vi "2D history.vi"   [LabVIEW 2021, in "Ring Buffer Strict Accessor Unit Tests.lvlib"]
uses:
  Ring Buffer Strict Accessor Unit Tests.lvlib
  Source/SubVIs/Endianess.ctl
  5a55b556-92d1-451c-b900-68450bc60f93.vi
  f229ef0f-1417-44bb-8496-cd9db5c3eb53.vi
  1447380f-0aa4-4579-b3fa-dda44ae90fdf.vi
  790f1047-96a1-4b40-bfa0-34b754fa4794.vi
  d13a2722-8c13-4299-92d3-41a30a9094d1.vi
  b8cc0c8d-ce30-4fd4-b064-991c88513f8d.vi
  ae355991-2fdf-4dcf-846e-4b605036bb22.vi
  1d5788e3-82fd-4730-bb71-cc7ffd3e5b8a.vi
  dea59858-e716-43e9-baf5-2617991b618f.vi
  5a55b556-92d1-451c-b900-68450bc60f93.vi/4c2a6c61-f100-483c-8a49-51e57025a24c.vi
  5a55b556-92d1-451c-b900-68450bc60f93.vi/e57bc314-87c7-4952-9bc8-929005dac297.vi
  <userlib>/bjustice/Ring Buffer for Time Series Data/API Poly.vi
  <userlib>/bjustice/Ring Buffer for Time Series Data/API/Write Array.vi
  f229ef0f-1417-44bb-8496-cd9db5c3eb53.vi/f2df9050-0eef-46c6-aff6-3ce3a8893ea5.vi
  1447380f-0aa4-4579-b3fa-dda44ae90fdf.vi/17d75e1a-130a-47e0-8f2c-6c7d90b8ca77.vi
  <userlib>/bjustice/Ring Buffer for Time Series Data/API/Read Full Rotated Buffer.vi
  Source/SubVIs/Search for time to keep.vi
  Source/SubVIs/Index ByteArray.vi
  1447380f-0aa4-4579-b3fa-dda44ae90fdf.vi/19bdd28a-0674-4be3-87bb-ec701e431d75.vi
  Source/SubVIs/error if empty buffer.vi
  790f1047-96a1-4b40-bfa0-34b754fa4794.vi/4c2a6c61-f100-483c-8a49-51e57025a24c.vi
  790f1047-96a1-4b40-bfa0-34b754fa4794.vi/e57bc314-87c7-4952-9bc8-929005dac297.vi
  d13a2722-8c13-4299-92d3-41a30a9094d1.vi/f2df9050-0eef-46c6-aff6-3ce3a8893ea5.vi
  b8cc0c8d-ce30-4fd4-b064-991c88513f8d.vi/17d75e1a-130a-47e0-8f2c-6c7d90b8ca77.vi
  b8cc0c8d-ce30-4fd4-b064-991c88513f8d.vi/19bdd28a-0674-4be3-87bb-ec701e431d75.vi
  ae355991-2fdf-4dcf-846e-4b605036bb22.vi/4c2a6c61-f100-483c-8a49-51e57025a24c.vi
  ae355991-2fdf-4dcf-846e-4b605036bb22.vi/e57bc314-87c7-4952-9bc8-929005dac297.vi
  1d5788e3-82fd-4730-bb71-cc7ffd3e5b8a.vi/f2df9050-0eef-46c6-aff6-3ce3a8893ea5.vi
  dea59858-e716-43e9-baf5-2617991b618f.vi/17d75e1a-130a-47e0-8f2c-6c7d90b8ca77.vi
  dea59858-e716-43e9-baf5-2617991b618f.vi/19bdd28a-0674-4be3-87bb-ec701e431d75.vi
  <userlib>/bjustice/Ring Buffer for Time Series Data/SubVIs/Split Values Array.vi
  <userlib>/bjustice/Ring Buffer for Time Series Data/SubVIs/Replace Values Array Multiple Timestamps.vi
  f229ef0f-1417-44bb-8496-cd9db5c3eb53.vi/f2df9050-0eef-46c6-aff6-3ce3a8893ea5.vi/63c583a5-c20f-4aba-9c90-661423dee4c4.vi
  f229ef0f-1417-44bb-8496-cd9db5c3eb53.vi/f2df9050-0eef-46c6-aff6-3ce3a8893ea5.vi/52385341-3d9c-45d2-aff5-e082a4793eb1.vi
  f229ef0f-1417-44bb-8496-cd9db5c3eb53.vi/f2df9050-0eef-46c6-aff6-3ce3a8893ea5.vi/37f29efa-f142-46b1-a185-f0098a95fbb6.vi
  f229ef0f-1417-44bb-8496-cd9db5c3eb53.vi/f2df9050-0eef-46c6-aff6-3ce3a8893ea5.vi/84b3d231-9afe-4b6e-afae-e0be43a31e4e.vi
  f229ef0f-1417-44bb-8496-cd9db5c3eb53.vi/f2df9050-0eef-46c6-aff6-3ce3a8893ea5.vi/c726271c-fc36-4bb7-8553-8945ec40c1cd.vi
  f229ef0f-1417-44bb-8496-cd9db5c3eb53.vi/f2df9050-0eef-46c6-aff6-3ce3a8893ea5.vi/a7b1d944-dc88-46f5-9d3e-305d46bbe1f6.vi
  f229ef0f-1417-44bb-8496-cd9db5c3eb53.vi/f2df9050-0eef-46c6-aff6-3ce3a8893ea5.vi/8abc4a6e-a1d2-4e85-879b-517e0ab55733.vi
  f229ef0f-1417-44bb-8496-cd9db5c3eb53.vi/f2df9050-0eef-46c6-aff6-3ce3a8893ea5.vi/bd347357-b475-4a03-9ac5-3b85ef11aecc.vi
  f229ef0f-1417-44bb-8496-cd9db5c3eb53.vi/f2df9050-0eef-46c6-aff6-3ce3a8893ea5.vi/391b36e9-a702-45e4-9499-3914f8833a58.vi
  f229ef0f-1417-44bb-8496-cd9db5c3eb53.vi/f2df9050-0eef-46c6-aff6-3ce3a8893ea5.vi/44155b33-c915-49ce-9e44-a66693aa70dd.vi
  f229ef0f-1417-44bb-8496-cd9db5c3eb53.vi/f2df9050-0eef-46c6-aff6-3ce3a8893ea5.vi/36977d53-dbe0-4dbc-b2ac-3dea4345b868.vi
  1447380f-0aa4-4579-b3fa-dda44ae90fdf.vi/17d75e1a-130a-47e0-8f2c-6c7d90b8ca77.vi/bbb64351-fa28-4ac1-b583-44e271193ecd.vi
  <userlib>/bjustice/Ring Buffer for Time Series Data/SubVIs/Rotate Buffer.vi
  Source/SubVIs/Search for oldest time to keep.vi
  Source/SubVIs/Search for newest time to keep.vi
  Source/SubVIs/datatype byte size.vi
  Source/SubVIs/array sizes to number of points.vi
  1447380f-0aa4-4579-b3fa-dda44ae90fdf.vi/19bdd28a-0674-4be3-87bb-ec701e431d75.vi/81c66277-30bd-484c-9c7c-9646f36721bb.vi
  1447380f-0aa4-4579-b3fa-dda44ae90fdf.vi/19bdd28a-0674-4be3-87bb-ec701e431d75.vi/7ca10173-70f1-4bfb-9c4b-948090662032.vi
  1447380f-0aa4-4579-b3fa-dda44ae90fdf.vi/19bdd28a-0674-4be3-87bb-ec701e431d75.vi/ea4aced9-3494-4b3f-b998-02af6afbdac4.vi
  1447380f-0aa4-4579-b3fa-dda44ae90fdf.vi/19bdd28a-0674-4be3-87bb-ec701e431d75.vi/022c581c-5349-49df-98f9-5a038829ee63.vi
  1447380f-0aa4-4579-b3fa-dda44ae90fdf.vi/19bdd28a-0674-4be3-87bb-ec701e431d75.vi/ed40bcc8-bbaa-4b61-9e1a-b4b75cf21b06.vi
  1447380f-0aa4-4579-b3fa-dda44ae90fdf.vi/19bdd28a-0674-4be3-87bb-ec701e431d75.vi/f4b703c2-aaab-40a0-b3da-b0c22dc82d50.vi
  1447380f-0aa4-4579-b3fa-dda44ae90fdf.vi/19bdd28a-0674-4be3-87bb-ec701e431d75.vi/1efa054f-b143-4d96-9f7e-584a7c6fa7fd.vi
  1447380f-0aa4-4579-b3fa-dda44ae90fdf.vi/19bdd28a-0674-4be3-87bb-ec701e431d75.vi/b7c29f3f-256a-4401-af9d-aa15374df391.vi
  1447380f-0aa4-4579-b3fa-dda44ae90fdf.vi/19bdd28a-0674-4be3-87bb-ec701e431d75.vi/2fb7b479-974d-4a18-8674-c4c8d9dc9a89.vi
  1447380f-0aa4-4579-b3fa-dda44ae90fdf.vi/19bdd28a-0674-4be3-87bb-ec701e431d75.vi/faac7175-5814-4bb6-a961-a8db1f460653.vi
  1447380f-0aa4-4579-b3fa-dda44ae90fdf.vi/19bdd28a-0674-4be3-87bb-ec701e431d75.vi/b6af2a6f-71a4-4cfe-837f-b196861458b0.vi
  d13a2722-8c13-4299-92d3-41a30a9094d1.vi/f2df9050-0eef-46c6-aff6-3ce3a8893ea5.vi/63c583a5-c20f-4aba-9c90-661423dee4c4.vi
  d13a2722-8c13-4299-92d3-41a30a9094d1.vi/f2df9050-0eef-46c6-aff6-3ce3a8893ea5.vi/52385341-3d9c-45d2-aff5-e082a4793eb1.vi
  d13a2722-8c13-4299-92d3-41a30a9094d1.vi/f2df9050-0eef-46c6-aff6-3ce3a8893ea5.vi/37f29efa-f142-46b1-a185-f0098a95fbb6.vi
  d13a2722-8c13-4299-92d3-41a30a9094d1.vi/f2df9050-0eef-46c6-aff6-3ce3a8893ea5.vi/84b3d231-9afe-4b6e-afae-e0be43a31e4e.vi
  d13a2722-8c13-4299-92d3-41a30a9094d1.vi/f2df9050-0eef-46c6-aff6-3ce3a8893ea5.vi/c726271c-fc36-4bb7-8553-8945ec40c1cd.vi
  d13a2722-8c13-4299-92d3-41a30a9094d1.vi/f2df9050-0eef-46c6-aff6-3ce3a8893ea5.vi/a7b1d944-dc88-46f5-9d3e-305d46bbe1f6.vi
  d13a2722-8c13-4299-92d3-41a30a9094d1.vi/f2df9050-0eef-46c6-aff6-3ce3a8893ea5.vi/8abc4a6e-a1d2-4e85-879b-517e0ab55733.vi
  d13a2722-8c13-4299-92d3-41a30a9094d1.vi/f2df9050-0eef-46c6-aff6-3ce3a8893ea5.vi/bd347357-b475-4a03-9ac5-3b85ef11aecc.vi
  d13a2722-8c13-4299-92d3-41a30a9094d1.vi/f2df9050-0eef-46c6-aff6-3ce3a8893ea5.vi/391b36e9-a702-45e4-9499-3914f8833a58.vi
  d13a2722-8c13-4299-92d3-41a30a9094d1.vi/f2df9050-0eef-46c6-aff6-3ce3a8893ea5.vi/44155b33-c915-49ce-9e44-a66693aa70dd.vi
  d13a2722-8c13-4299-92d3-41a30a9094d1.vi/f2df9050-0eef-46c6-aff6-3ce3a8893ea5.vi/36977d53-dbe0-4dbc-b2ac-3dea4345b868.vi
  b8cc0c8d-ce30-4fd4-b064-991c88513f8d.vi/17d75e1a-130a-47e0-8f2c-6c7d90b8ca77.vi/bbb64351-fa28-4ac1-b583-44e271193ecd.vi
  b8cc0c8d-ce30-4fd4-b064-991c88513f8d.vi/19bdd28a-0674-4be3-87bb-ec701e431d75.vi/81c66277-30bd-484c-9c7c-9646f36721bb.vi
  b8cc0c8d-ce30-4fd4-b064-991c88513f8d.vi/19bdd28a-0674-4be3-87bb-ec701e431d75.vi/7ca10173-70f1-4bfb-9c4b-948090662032.vi
  b8cc0c8d-ce30-4fd4-b064-991c88513f8d.vi/19bdd28a-0674-4be3-87bb-ec701e431d75.vi/ea4aced9-3494-4b3f-b998-02af6afbdac4.vi
  b8cc0c8d-ce30-4fd4-b064-991c88513f8d.vi/19bdd28a-0674-4be3-87bb-ec701e431d75.vi/022c581c-5349-49df-98f9-5a038829ee63.vi
  b8cc0c8d-ce30-4fd4-b064-991c88513f8d.vi/19bdd28a-0674-4be3-87bb-ec701e431d75.vi/ed40bcc8-bbaa-4b61-9e1a-b4b75cf21b06.vi
  b8cc0c8d-ce30-4fd4-b064-991c88513f8d.vi/19bdd28a-0674-4be3-87bb-ec701e431d75.vi/f4b703c2-aaab-40a0-b3da-b0c22dc82d50.vi
  b8cc0c8d-ce30-4fd4-b064-991c88513f8d.vi/19bdd28a-0674-4be3-87bb-ec701e431d75.vi/1efa054f-b143-4d96-9f7e-584a7c6fa7fd.vi
  b8cc0c8d-ce30-4fd4-b064-991c88513f8d.vi/19bdd28a-0674-4be3-87bb-ec701e431d75.vi/b7c29f3f-256a-4401-af9d-aa15374df391.vi
  b8cc0c8d-ce30-4fd4-b064-991c88513f8d.vi/19bdd28a-0674-4be3-87bb-ec701e431d75.vi/2fb7b479-974d-4a18-8674-c4c8d9dc9a89.vi
  b8cc0c8d-ce30-4fd4-b064-991c88513f8d.vi/19bdd28a-0674-4be3-87bb-ec701e431d75.vi/faac7175-5814-4bb6-a961-a8db1f460653.vi
  b8cc0c8d-ce30-4fd4-b064-991c88513f8d.vi/19bdd28a-0674-4be3-87bb-ec701e431d75.vi/b6af2a6f-71a4-4cfe-837f-b196861458b0.vi
  1d5788e3-82fd-4730-bb71-cc7ffd3e5b8a.vi/f2df9050-0eef-46c6-aff6-3ce3a8893ea5.vi/63c583a5-c20f-4aba-9c90-661423dee4c4.vi
  1d5788e3-82fd-4730-bb71-cc7ffd3e5b8a.vi/f2df9050-0eef-46c6-aff6-3ce3a8893ea5.vi/52385341-3d9c-45d2-aff5-e082a4793eb1.vi
  1d5788e3-82fd-4730-bb71-cc7ffd3e5b8a.vi/f2df9050-0eef-46c6-aff6-3ce3a8893ea5.vi/37f29efa-f142-46b1-a185-f0098a95fbb6.vi
  1d5788e3-82fd-4730-bb71-cc7ffd3e5b8a.vi/f2df9050-0eef-46c6-aff6-3ce3a8893ea5.vi/84b3d231-9afe-4b6e-afae-e0be43a31e4e.vi
  1d5788e3-82fd-4730-bb71-cc7ffd3e5b8a.vi/f2df9050-0eef-46c6-aff6-3ce3a8893ea5.vi/c726271c-fc36-4bb7-8553-8945ec40c1cd.vi
  1d5788e3-82fd-4730-bb71-cc7ffd3e5b8a.vi/f2df9050-0eef-46c6-aff6-3ce3a8893ea5.vi/a7b1d944-dc88-46f5-9d3e-305d46bbe1f6.vi
  1d5788e3-82fd-4730-bb71-cc7ffd3e5b8a.vi/f2df9050-0eef-46c6-aff6-3ce3a8893ea5.vi/8abc4a6e-a1d2-4e85-879b-517e0ab55733.vi
  1d5788e3-82fd-4730-bb71-cc7ffd3e5b8a.vi/f2df9050-0eef-46c6-aff6-3ce3a8893ea5.vi/bd347357-b475-4a03-9ac5-3b85ef11aecc.vi
  1d5788e3-82fd-4730-bb71-cc7ffd3e5b8a.vi/f2df9050-0eef-46c6-aff6-3ce3a8893ea5.vi/391b36e9-a702-45e4-9499-3914f8833a58.vi
  1d5788e3-82fd-4730-bb71-cc7ffd3e5b8a.vi/f2df9050-0eef-46c6-aff6-3ce3a8893ea5.vi/44155b33-c915-49ce-9e44-a66693aa70dd.vi
  1d5788e3-82fd-4730-bb71-cc7ffd3e5b8a.vi/f2df9050-0eef-46c6-aff6-3ce3a8893ea5.vi/36977d53-dbe0-4dbc-b2ac-3dea4345b868.vi
  dea59858-e716-43e9-baf5-2617991b618f.vi/17d75e1a-130a-47e0-8f2c-6c7d90b8ca77.vi/bbb64351-fa28-4ac1-b583-44e271193ecd.vi
  dea59858-e716-43e9-baf5-2617991b618f.vi/19bdd28a-0674-4be3-87bb-ec701e431d75.vi/81c66277-30bd-484c-9c7c-9646f36721bb.vi
  dea59858-e716-43e9-baf5-2617991b618f.vi/19bdd28a-0674-4be3-87bb-ec701e431d75.vi/7ca10173-70f1-4bfb-9c4b-948090662032.vi
  dea59858-e716-43e9-baf5-2617991b618f.vi/19bdd28a-0674-4be3-87bb-ec701e431d75.vi/ea4aced9-3494-4b3f-b998-02af6afbdac4.vi
  dea59858-e716-43e9-baf5-2617991b618f.vi/19bdd28a-0674-4be3-87bb-ec701e431d75.vi/022c581c-5349-49df-98f9-5a038829ee63.vi
  dea59858-e716-43e9-baf5-2617991b618f.vi/19bdd28a-0674-4be3-87bb-ec701e431d75.vi/ed40bcc8-bbaa-4b61-9e1a-b4b75cf21b06.vi
  dea59858-e716-43e9-baf5-2617991b618f.vi/19bdd28a-0674-4be3-87bb-ec701e431d75.vi/f4b703c2-aaab-40a0-b3da-b0c22dc82d50.vi
  dea59858-e716-43e9-baf5-2617991b618f.vi/19bdd28a-0674-4be3-87bb-ec701e431d75.vi/1efa054f-b143-4d96-9f7e-584a7c6fa7fd.vi
  dea59858-e716-43e9-baf5-2617991b618f.vi/19bdd28a-0674-4be3-87bb-ec701e431d75.vi/b7c29f3f-256a-4401-af9d-aa15374df391.vi
  dea59858-e716-43e9-baf5-2617991b618f.vi/19bdd28a-0674-4be3-87bb-ec701e431d75.vi/2fb7b479-974d-4a18-8674-c4c8d9dc9a89.vi
  dea59858-e716-43e9-baf5-2617991b618f.vi/19bdd28a-0674-4be3-87bb-ec701e431d75.vi/faac7175-5814-4bb6-a961-a8db1f460653.vi
  dea59858-e716-43e9-baf5-2617991b618f.vi/19bdd28a-0674-4be3-87bb-ec701e431d75.vi/b6af2a6f-71a4-4cfe-837f-b196861458b0.vi
  <userlib>/bjustice/Ring Buffer for Time Series Data/SubVIs/Enforce array size multiple timestamps.vi
  Source/API/New.vi
  <vilib>/Utility/error.llb/Error Cluster From Error Code.vi
  <vilib>/Utility/error.llb/Trim Whitespace.vi
  <vilib>/addons/_JKI Toolkits/Caraya/classes/Assert/Assert True.vi
  <vilib>/addons/_JKI Toolkits/Caraya/classes/Assert/Assert Not Error.vi
  <vilib>/addons/_JKI Toolkits/Caraya/classes/Assert/Assert Equal Value_Variant.vi
  Source/Ring Buffer Strict Accessor.lvlib
  <vilib>/addons/_JKI Toolkits/Caraya/classes/Assert/Assert.lvclass
  <vilib>/addons/_JKI Toolkits/Caraya/classes/Test/Test.lvclass
types:
  T1 = typedef "Ring Buffer Strict Accessor.lvlib/Endianess.ctl" = enum16{"big-endian", "little-endian"}
  T2 = typedef "Ring Buffer Strict Accessor.lvlib/RingBufferHandle.ctl" = cluster{"Ring buffer DVR":refnum<data-value>, "Data Type":T3, "Size(s)":i32[], "Endianess":T1, "Buffer Size (#timestamps) [init]":i32}
  T3 = typedef "Ring Buffer Strict Accessor.lvlib/DataType.ctl" = enum16{"uint8", "uint16", "uint32", "uint64", "int8", "int16", "int32", "int64", "float", "double", "extended"}
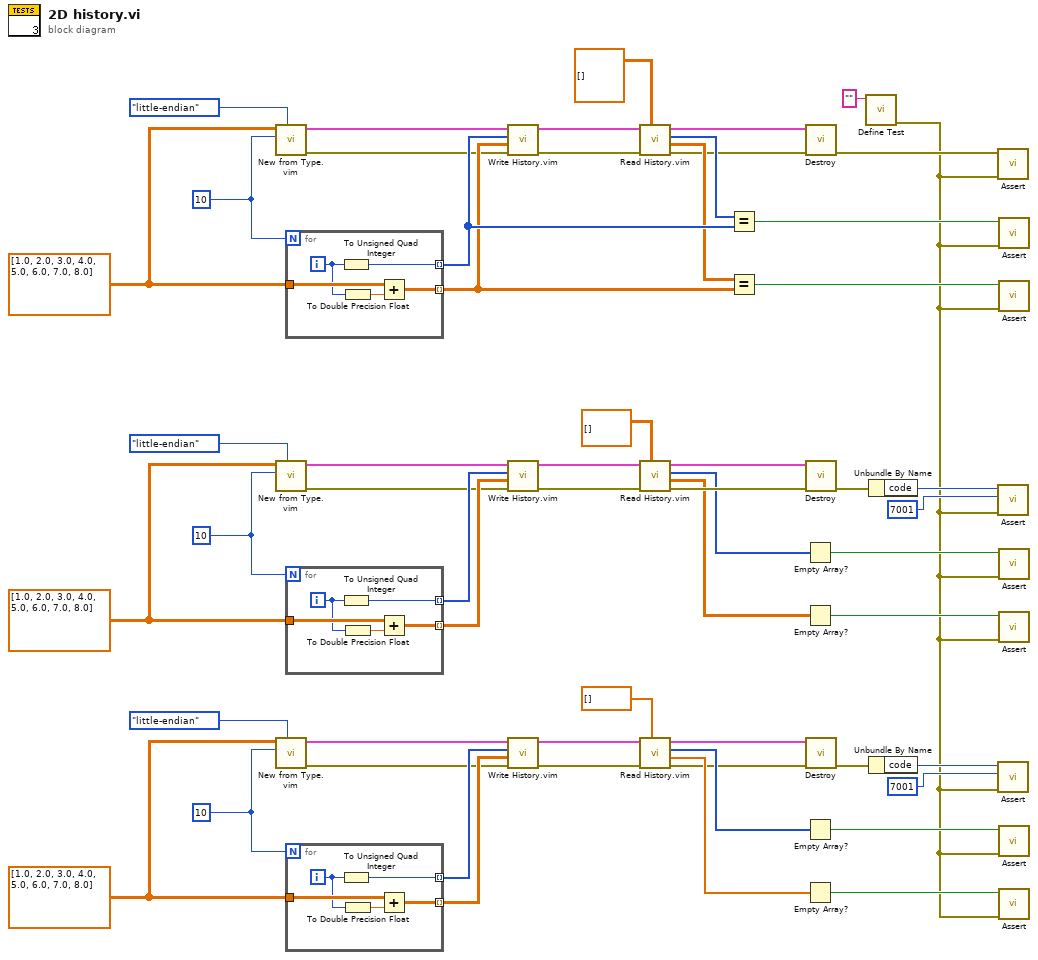
[diagram p0: block diagram]
diagram:
  w2 = 10 ("Buffer Size (#timestamps)")
  w3 = dbl[][] [[1.0, 2.0, 3.0, 4.0], [5.0, 6.0, 7.0, 8.0]]
  w6 = 10 ("Buffer Size (#timestamps)")
  w7 = dbl[][] [[1.0, 2.0, 3.0, 4.0], [5.0, 6.0, 7.0, 8.0]]
  w12 = 10 ("Buffer Size (#timestamps)")
  w13 = dbl[][] [[1.0, 2.0, 3.0, 4.0], [5.0, 6.0, 7.0, 8.0]]
  n1 = call "New from Type.vim"("Endianess"=Endianess."little-endian", "Buffer Size (#timestamps)"=w12, "LV type (array size cannot be empty)"=w13) -> ("error out"=w14:errorcluster, "Ring Buffer"=w15:T2)  [unwired: 7 in]
  n2 = call "New from Type.vim"("Endianess"=Endianess."little-endian", "Buffer Size (#timestamps)"=w6, "LV type (array size cannot be empty)"=w7) -> ("error out"=w9:errorcluster, "Ring Buffer"=w10:T2)  [unwired: 7 in]
  n3 = call "New from Type.vim"("Endianess"=Endianess."little-endian", "Buffer Size (#timestamps)"=w2, "LV type (array size cannot be empty)"=w3) -> ("error out"=w4:errorcluster, "Ring Buffer"=w5:T2)  [unwired: 7 in]
  n4 = for {
    N: w12 -> [_]
    tunnel: w13 -> [w62]
    tunnel: [w61] -> w51 mode=indexing
    tunnel: [w60] -> w53 mode=indexing
    i -> [w59]
    n5 = To Unsigned Quad Integer(1:w59) -> (0:w60:u64)
    n6 = To Double Precision Float(number=w59) -> (double precision float=w58:dbl)
    n7 = Add(x=w62, y=w58) -> (x+y=w61:dbl[][])
  }
  n8 = for {
    N: w6 -> [_]
    tunnel: w7 -> [w67]
    tunnel: [w66] -> w44 mode=indexing
    tunnel: [w65] -> w43 mode=indexing
    i -> [w64]
    n9 = To Unsigned Quad Integer(1:w64) -> (0:w65:u64)
    n10 = To Double Precision Float(number=w64) -> (double precision float=w63:dbl)
    n11 = Add(x=w67, y=w63) -> (x+y=w66:dbl[][])
  }
  n12 = for {
    N: w2 -> [_]
    tunnel: w3 -> [w72]
    tunnel: [w71] -> w19 mode=indexing
    tunnel: [w70] -> w20 mode=indexing
    i -> [w69]
    n13 = To Unsigned Quad Integer(1:w69) -> (0:w70:u64)
    n14 = To Double Precision Float(number=w69) -> (double precision float=w68:dbl)
    n15 = Add(x=w72, y=w68) -> (x+y=w71:dbl[][])
  }
  n16 = call "Write History.vim"("error in (no error)"=w14, "LV DataType"=w51, "Timestamps"=w53, "Ring Buffer"=w15) -> ("error out"=w50:errorcluster, "Ring Buffer"=w57:T2)  [unwired: 6 in]
  n17 = call "Write History.vim"("error in (no error)"=w9, "LV DataType"=w44, "Timestamps"=w43, "Ring Buffer"=w10) -> ("error out"=w45:errorcluster, "Ring Buffer"=w40:T2)  [unwired: 6 in]
  n18 = call "Write History.vim"("error in (no error)"=w4, "LV DataType"=w19, "Timestamps"=w20, "Ring Buffer"=w5) -> ("error out"=w18:errorcluster, "Ring Buffer"=w23:T2)  [unwired: 6 in]
  n19 = call "Read History.vim"("data type"=dbl[][][] [], "error in (no error)"=w50, "Ring Buffer"=w57) -> ("error out"=w49:errorcluster, "Values"=w52:dbl[][][], "Timestamps"=w54:u64[], "Ring Buffer"=w56:T2)  [unwired: 5 in]
  n20 = call "Read History.vim"("data type"=dbl[][] [], "error in (no error)"=w45, "Ring Buffer"=w40) -> ("error out"=w46:errorcluster, "Values"=w33:dbl[][], "Timestamps"=w34:u64[], "Ring Buffer"=w41:T2)  [unwired: 5 in]
  n21 = call "Read History.vim"("data type"=dbl[] [], "error in (no error)"=w18, "Ring Buffer"=w23) -> ("error out"=w17:errorcluster, "Values"=w28:dbl[], "Timestamps"=w27:u64[], "Ring Buffer"=w22:T2)  [unwired: 5 in]
  n22 = Equal?(x=w54, y=w53) -> (x = y?=w48:bool)
  n23 = Equal?(x=w52, y=w51) -> (x = y?=w47:bool)
  n24 = Empty Array?(array=w34) -> (empty?=w32:bool)
  n25 = Empty Array?(array=w33) -> (empty?=w31:bool)
  n26 = Empty Array?(array=w27) -> (empty?=w29:bool)
  n27 = Empty Array?(array=w28) -> (empty?=w30:bool)
  n28 = call "Destroy.vi"("error in (no error)"=w49, "Ring Buffer"=w56) -> ("error out"=w39:errorcluster)  [unwired: 9 in]
  n29 = call "Destroy.vi"("error in (no error)"=w46, "Ring Buffer"=w41) -> ("error out"=w37:errorcluster)  [unwired: 9 in]
  n30 = call "Destroy.vi"("error in (no error)"=w17, "Ring Buffer"=w22) -> ("error out"=w24:errorcluster)  [unwired: 9 in]
  n31 = call <vilib>:"Define Test.vi"("Label (VI Title)"="") -> ("error out"=w16:errorcluster)  [unwired: 9 in, 1 out]
  n32 = Unbundle By Name(w37) -> ("code"=w36:i32)
  n33 = Unbundle By Name(w24) -> ("code"=w25:i32)
  n34 = call-poly <vilib>:"Assert.vi"("error in (no error)"=w16, "Not Error?"=w39) -> ()  [unwired: 8 in, 2 out]
  n35 = call-poly <vilib>:"Assert.vi"("error in (no error)"=w16, "Y"=7001 ("code"), "X"=w36) -> ()  [unwired: 7 in, 2 out]
  n36 = call-poly <vilib>:"Assert.vi"("error in (no error)"=w16, "Y"=7001 ("code"), "X"=w25) -> ()  [unwired: 7 in, 2 out]
  n37 = call-poly <vilib>:"Assert.vi"("error in (no error)"=w16, "True?"=w48) -> ()  [unwired: 8 in, 2 out]
  n38 = call-poly <vilib>:"Assert.vi"("error in (no error)"=w16, "True?"=w47) -> ()  [unwired: 8 in, 2 out]
  n39 = call-poly <vilib>:"Assert.vi"("error in (no error)"=w16, "True?"=w32) -> ()  [unwired: 8 in, 2 out]
  n40 = call-poly <vilib>:"Assert.vi"("error in (no error)"=w16, "True?"=w31) -> ()  [unwired: 8 in, 2 out]
  n41 = call-poly <vilib>:"Assert.vi"("error in (no error)"=w16, "True?"=w29) -> ()  [unwired: 8 in, 2 out]
  n42 = call-poly <vilib>:"Assert.vi"("error in (no error)"=w16, "True?"=w30) -> ()  [unwired: 8 in, 2 out]
